vi "Visualizacion_NEW.vi"() -> ()   [LabVIEW 2021]
uses:
  <vilib>/Modbus/master/Modbus Master.lvclass
  <vilib>/Modbus/master/Create Master Instance (TCP).vi
panel:
  out "MEAN (T)":sgl format="%0.2f"
  out "Peltiers enable":bool
  out "Program Status":bool
  out "SP (T)":sgl
  out "Segmento_temp":u16
  in  "?":T1(tab)
  in  "?":T2(tab)
  out "TEMPERATURA MEDIA":dynamicdata(graph)
  out "ALL TOGETHER":dynamicdata(graph)
  out "VALVULA 1 Y BOBINA 1":dynamicdata(graph)
  out "VALVULA 2 Y BOBINA 2":dynamicdata(graph)
  out "VALVULA 3 Y BOBINA 3":dynamicdata(graph)
  out "VALVULA 4 Y BOBINA 4":dynamicdata(graph)
  out "VALVULA 5  Y BOBINA 5":dynamicdata(graph)
  out "VALVULA 6 Y BOBINA 6":dynamicdata(graph)
  out "VALVULA 7 Y BOBINA 7":dynamicdata(graph)
  out "VALVULA 8 Y PELTIER 8":dynamicdata(graph)
  out "Camara climatica":dynamicdata(graph)
  out "current time":timestamp
  out "W1.16":bool
  out "W1.15":bool
  out "W1.11":bool
  out "1.10":bool
  out "W1.14":bool
  out "W1.13":bool
  out "W1.12":bool
  out "W1.1":bool
  out "W2":bool
  out "W3":bool
  out "W4":bool
  out "W1.2":bool
  out "W1.3":bool
  out "W1.6":bool
  out "W1.5":bool
  out "W1.4":bool
  out "W1.9":bool
  out "W1.8":bool
  out "W1.7":bool
  out "warnings table":T3(array[cluster]) {"Time Stamp" format="%<%.3X %x>T"}
  in  "Reset":bool
  out "Comunicacion Modbus":errorcluster
  in  "Digital Input Bitron Simulation":bool
  in  "Pelt ºC/min":dbl=2.5
  in  "Cam ºC/min":dbl=2.2
  in  "Tiempo máximo de ciclo(min)":dbl=90.0
  in  "Setpoint corte frío(ºC)":dbl=-30.0
  in  "Setpoint Frío(ºC)":dbl=-40.0
  in  "Setpoint peltiers(ºC)":dbl=85.0
  in  "Tiempo estabilidad de Frío(min)":dbl=15.0
  in  "Tiempo mínimo de ciclo(min)":dbl=70.0
  in  "Setpoint calor corte rampa(ºC)":dbl=51.0
  in  "T ciclo (Bitron FSM Sim)":dbl=90.0
  in  "Setpoint calor cam":dbl=55.0
  in  "Save Parameters":bool
  in  "PWM 4(SP)":u16
  in  "PWM 3(SP) 2":u16
  in  "PWM 2(SP) 2":u16
  in  "PWM 1(SP) 2":u16
  in  "PWM 8(SP)":u16
  in  "PWM 7(SP)":u16
  in  "PWM 6(SP)":u16
  in  "PWM 5(SP)":u16
  in  "Test PWM (%)":bool
  in  "Conf PIDs":bool
  in  "TestPID 8(ºC)":u16
  in  "TestPID 4(ºC)":u16
  in  "TestPID3(ºC)":u16
  in  "TestPID 2(ºC)":u16
  in  "TestPID 1(ºC)":u16
  in  "TestPID 5(ºC)":u16
  in  "TestPID 6(ºC)":u16
  in  "TestPID 7(ºC)":u16
  out "Temp Man 2":sgl
  out "PWM 1(SP)":u16
  out "Temp Man 3":sgl format="%#.2g"
  out "Temp Man 1":sgl format="%#.2g"
  out "Temp Man 4":sgl
  out "PWM 2(SP)":u16
  out "Temp Man 5":sgl format="%#.2g"
  out "PWM 3(SP)":u16
  out "PWM 4(SP)":u16
  out "Temp Man 6":sgl
  out "Temp Man 7":sgl format="%#.2g"
  out "Temp Man 8":sgl
  out "PWM 6(SP)":u16
  out "PWM 7(SP)":u16
  out "PWM 5(SP)":u16
  out "PWM 8(SP)":u16
  out "Temp bob 1":sgl
  out "Temp bob 2":sgl
  out "Temp bob 3":sgl format="%#.2g"
  out "Temp bob 6":sgl
  out "Temp bob 7":sgl format="%#.2g"
  out "Temp bob 8":sgl
  in  "Enable PI 5":bool
  in  "Enable PI 6":bool=TRUE
  in  "Enable PI 7":bool
  in  "Enable PI 8":bool
  out "Temp bob 5":sgl format="%#.2g"
  in  "Descarte Media Temps":u16=1 max=3 step=1
  out "Temp bob 4":sgl
  in  "Enable PI 1":bool
  in  "Enable PI 2":bool
  in  "Enable PI 3":bool
  in  "Enable PI 4":bool=TRUE
  in  "Test PID (ºC)":bool
  in  "Tiempo de guardado":u32=600
  out "data to be saved":dbl[][](array[numeric])
  out "Guardando en disco":bool
  out "array w/ subset deleted":dbl[][](array[numeric])
  out "size(s)":i32
  out "W to save":string[][](array[string])
  in  "Warning saved":bool
  in  "Tiempo/dato (s)":u32=1
  out "DO H2 Lab":bool
  in  "Guardar datos":bool=TRUE
  out "senal_bitron":bool
  in  "Stop Control Program":bool
  out "Coils write":bool[](array[boolean])
  out "Int values":u16[](array[numeric])
  out "SGL values":sgl[](array[numeric])
  out "coil values":bool[](array[boolean])
  out "ComunicacionCRIO":bool
  in  "run_program":bool
  out "Setpoint_temp_write":dbl
  out "Setpoint_hum_write":dbl
  out "Temperatura Camara":dbl
  out "Humedad relativa (HR)":dbl
  in  "Pause_Entrar_camara":bool
  in  "Pause":bool
  in  "stop":bool
  in  "Tab Control":T4(tab)
  out "T Man 5":dbl(slide) scale=-45.0..90.0
  out "T Man 1":dbl(slide) scale=-45.0..90.0
  out "T Man 2":dbl(slide) scale=-45.0..90.0
  out "T Man 3":dbl(slide) scale=-45.0..90.0
  out "T Man 4":dbl(slide) scale=-45.0..90.0
  out "T Man 6":dbl(slide) scale=-45.0..90.0
  out "T Man 7":dbl(slide) scale=-45.0..90.0
  out "T Man 8":dbl(slide) scale=-45.0..90.0
  out "T bob 5":dbl(slide) scale=-45.0..95.0
  out "T bob 1":dbl(slide) scale=-45.0..95.0
  out "T bob 2":dbl(slide) scale=-45.0..95.0
  out "T bob 3":dbl(slide) scale=-45.0..95.0
  out "T bob 4":dbl(slide) scale=-45.0..95.0
  out "T bob 6":dbl(slide) scale=-45.0..95.0
  out "T bob 7":dbl(slide) scale=-45.0..95.0
  out "T bob 8":dbl(slide) scale=-45.0..95.0
  # "Control Programa Principal"
  # "Cámara climática"
  # "ºC"
  # "ºC"
  # "%"
  # "%"
  # "Simulación señal Bitron"
  # "ºC"
  # "HR"
  # "TempCC"
  # "SP_HR"
  # "SP_TempCC"
  # "Mean T"
  # "Warnings y Errores"
  # "Parametros y configuracion para la curva de ciclado"
  # "ºC"
  # "ºC"
  # "VALVE 4"
  # "VALVE 8"
  # "%"
  # "%"
  # "ºC"
  # "ºC"
  # "ºC"
  # "ºC"
  # "VALVE 3"
  # "%"
  # "%"
  # "VALVE 7"
  # "ºC"
  # "ºC"
  # "ºC"
  # "ºC"
  # "VALVE 2"
  # "%"
  # "%"
  # "VALVE 6"
  # "ºC"
  # "ºC"
  # "ºC"
  # "ºC"
  # "VALVE 1"
  # "%"
  # "%"
  # "VALVE 5"
  # "ºC"
  # "ºC"
  # "1 Dato\n----------------"
  # "Frecuencia de guardado:"
  # "s"
  # "s"
  # "T Manifolds:"
  # "1               2               3               4               5               6               7               8"
  # "T Bobinas:"
  # "1               2               3               4               5                 6               7               8"
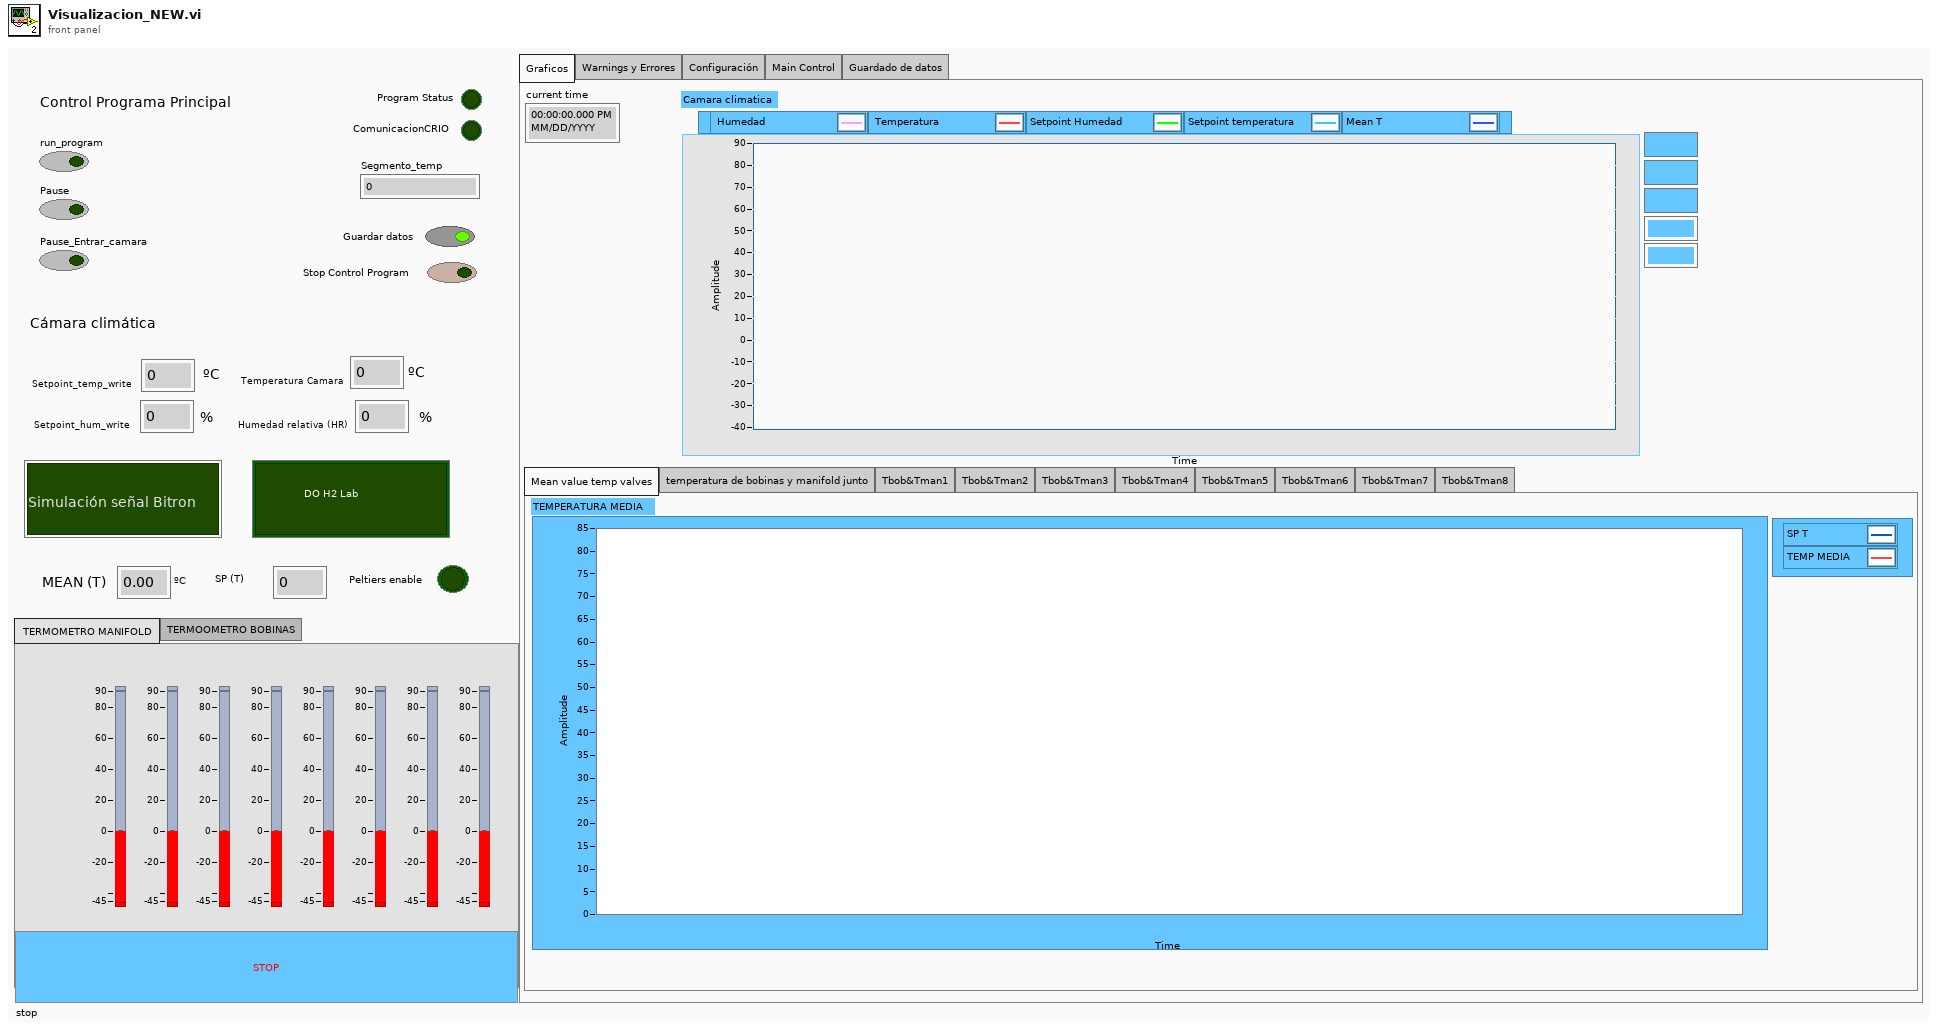
[diagram p1: front panel]
types:
  T1 = enum32{"Graficos", "Warnings y Errores", "Configuración", "Main Control", "Guardado de datos"}
  T2 = enum32{"Mean value temp valves", "temperatura de bobinas y manifold junto", "Tbob&Tman1", "Tbob&Tman2", "Tbob&Tman3", "Tbob&Tman4", "Tbob&Tman5", "Tbob&Tman6", "Tbob&Tman7", "Tbob&Tman8"}
  T3 = cluster{"Time Stamp":timestamp, "Descripcion":string, "Numeric":i32}[]
  T4 = enum32{"TERMOMETRO MANIFOLD ", "TERMOOMETRO BOBINAS"}
  T5 = enum8{"Enabled", "Disabled", "Disabled and Grayed Out"}
  T6 = enum16{"open", "open or create", "create or replace", "create", "open (read-only)"}
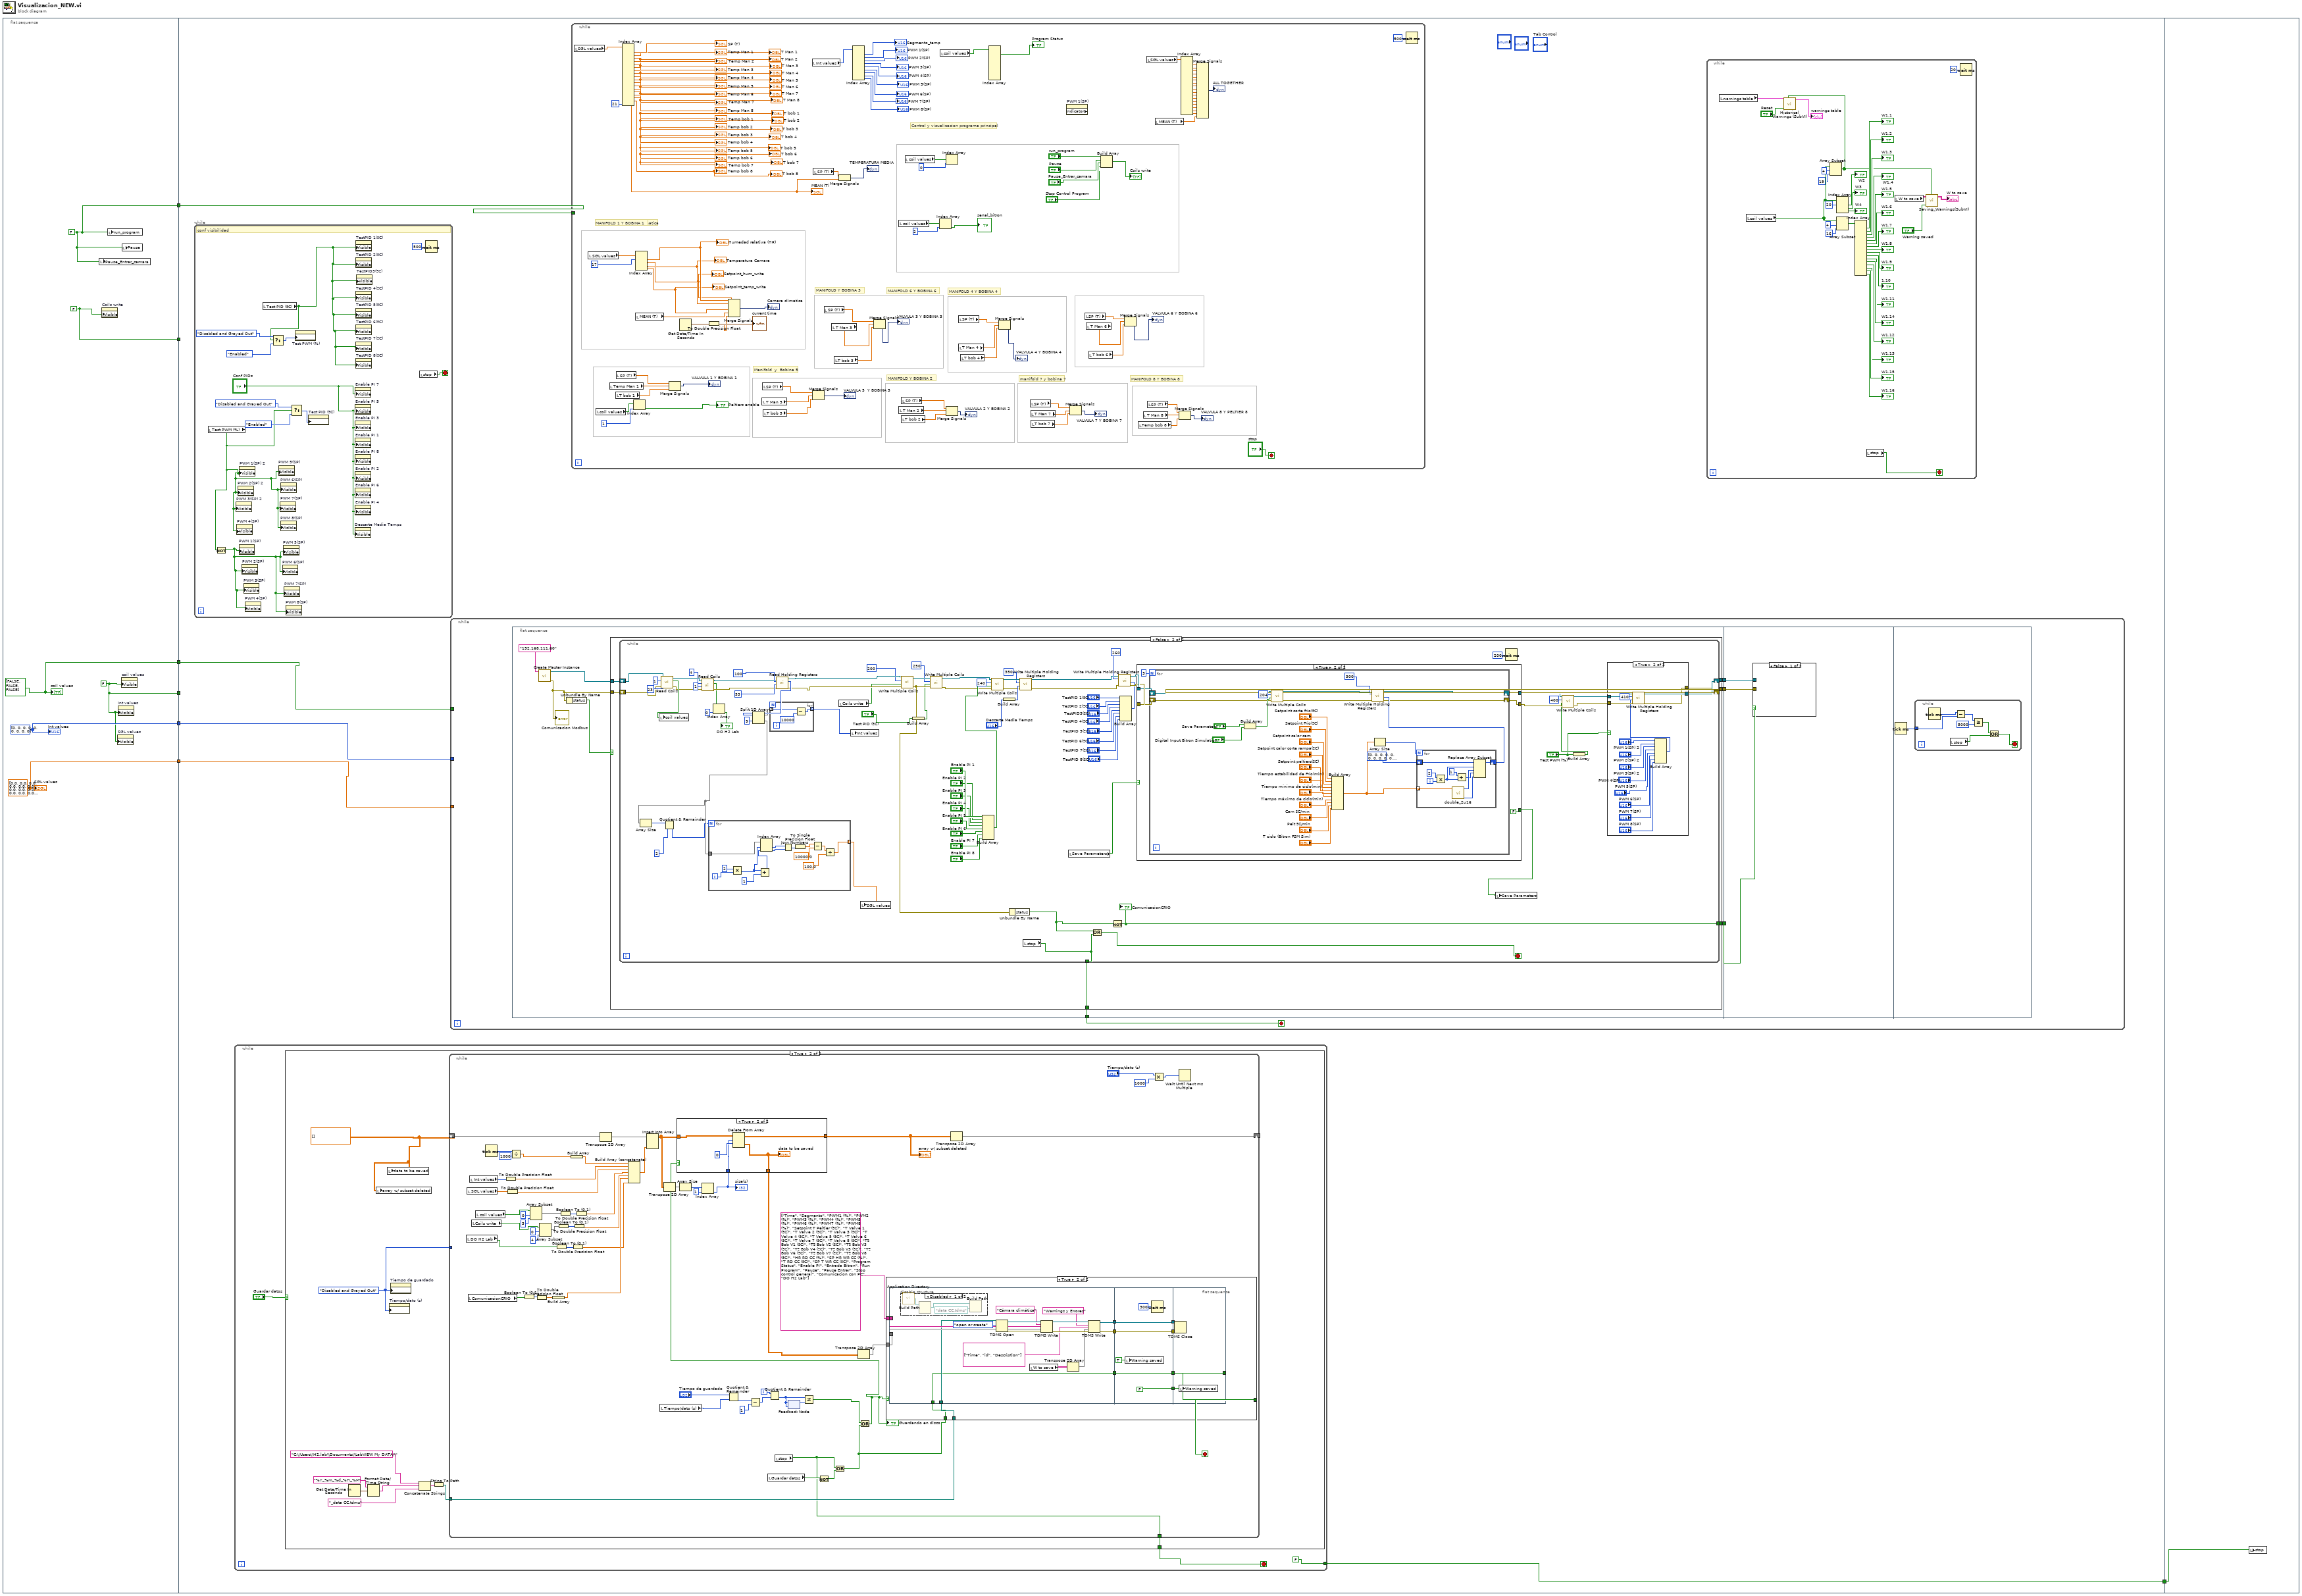
[diagram p0: block diagram]
diagram:
  n1 = flat-sequence {
    tunnel: [w13] -> w7
    tunnel: [w12] -> w6
    tunnel: [w11] -> w5
    tunnel: [w10] -> w4
    tunnel: [w8] -> w2
    tunnel: [w9] -> w1
    tunnel: w7 -> [w18]
    tunnel: w6 -> [w17]
    tunnel: w5 -> [w16]
    tunnel: w4 -> [w15]
    tunnel: [w14] -> w3
    tunnel: w2 -> [_]
    tunnel: w1 -> [_]
    tunnel: w3 -> [w501]
    frame #0 {
      w9 = FALSE ("Visible")
      w8 = FALSE ("Visible")
      w11 = sgl[] [0.0, 0.0, 0.0, 0.0, 0.0, 0.0, 0.0, 0.0, 0.0, 0.0, 0.0, 0.0, 0.0, 0.0, 0.0, 0.0, 0.0, 0.0, 0.0, 0.0, 0.0] ("SGL values")
      w12 = u16[] [0, 0, 0, 0, 0, 0, 0, 0, 0] ("Int values")
      w10 = FALSE ("run_program")
      w13 = bool[] [FALSE, FALSE, FALSE] ("coil values")
      n2 = local write "Pause_Entrar_camara"(w10) -> ()
      n3 = property on="Coils write" class="Arr (strict)"("Visible"=w9) -> ()  [unwired: 2 in, 2 out]
      n4 = local write "run_program"(w10) -> ()
      n5 = property on="SGL values" class="Arr (strict)"("Visible"=w8) -> ()  [unwired: 2 in, 2 out]
      n6 = property on="Int values" class="Arr (strict)"("Visible"=w8) -> ()  [unwired: 2 in, 2 out]
      n7 = property on="coil values" class="Arr (strict)"("Visible"=w8) -> ()  [unwired: 2 in, 2 out]
      n8 = local write "Pause"(w10) -> ()
      "coil values" <- w13
      "Int values" <- w12
      "SGL values" <- w11
    }
    frame #1 {
      n9 = while {
        stop <- w30 stop-if-true
        # "conf visibilidad"
        n10 = local read "Test PWM (%)"() -> (w19:bool)
        n11 = Not(x=w19) -> (.not. x?=w27:bool)
        n12 = property on="PWM 3(SP) 2" class="DigNum (strict)"("Visible"=w19) -> ()  [unwired: 2 in, 2 out]
        n13 = property on="PWM 4(SP)" class="DigNum (strict)"("Visible"=w19) -> ()  [unwired: 2 in, 2 out]
        n14 = property on="PWM 2(SP) 2" class="DigNum (strict)"("Visible"=w19) -> ()  [unwired: 2 in, 2 out]
        n15 = property on="PWM 1(SP)" class="DigNum (strict)"("Visible"=w27) -> ()  [unwired: 2 in, 2 out]
        n16 = property on="PWM 1(SP) 2" class="DigNum (strict)"("Visible"=w19) -> ()  [unwired: 2 in, 2 out]
        n17 = property on="PWM 2(SP)" class="DigNum (strict)"("Visible"=w27) -> ()  [unwired: 2 in, 2 out]
        n18 = property on="PWM 3(SP)" class="DigNum (strict)"("Visible"=w27) -> ()  [unwired: 2 in, 2 out]
        n19 = property on="PWM 4(SP)" class="DigNum (strict)"("Visible"=w27) -> ()  [unwired: 2 in, 2 out]
        n20 = local read "Test PID (ºC)"() -> (w23:bool)
        n21 = Select(t=T5."Disabled and Grayed Out" ("Disabled"), s=w23, f=T5."Enabled" ("Disabled")) -> (s? t:f=w24:T5)
        n22 = property on="PWM 5(SP)" class="DigNum (strict)"("Visible"=w19) -> ()  [unwired: 2 in, 2 out]
        n23 = property on="PWM 7(SP)" class="DigNum (strict)"("Visible"=w19) -> ()  [unwired: 2 in, 2 out]
        n24 = property on="PWM 6(SP)" class="DigNum (strict)"("Visible"=w19) -> ()  [unwired: 2 in, 2 out]
        n25 = property on="PWM 8(SP)" class="DigNum (strict)"("Visible"=w19) -> ()  [unwired: 2 in, 2 out]
        n26 = property on="PWM 6(SP)" class="DigNum (strict)"("Visible"=w27) -> ()  [unwired: 2 in, 2 out]
        n27 = property on="PWM 5(SP)" class="DigNum (strict)"("Visible"=w27) -> ()  [unwired: 2 in, 2 out]
        n28 = property on="PWM 7(SP)" class="DigNum (strict)"("Visible"=w27) -> ()  [unwired: 2 in, 2 out]
        n29 = property on="PWM 8(SP)" class="DigNum (strict)"("Visible"=w27) -> ()  [unwired: 2 in, 2 out]
        n30 = Select(t=T5."Disabled and Grayed Out" ("Disabled"), s=w19, f=T5."Enabled" ("Disabled")) -> (s? t:f=w20:T5)
        n31 = property on="Test PWM (%)" class="Bool (strict)"("DisabledEnum"=w24) -> ()  [unwired: 2 in, 2 out]
        n32 = property on="Test PID (ºC)" class="Bool (strict)"("DisabledEnum"=w20) -> ()  [unwired: 2 in, 2 out]
        n33 = property on="Descarte Media Temps" class="DigNum (strict)"("Visible"="Conf PIDs") -> ()  [unwired: 2 in, 2 out]
        n34 = property on="Enable PI 7" class="Bool (strict)"("Visible"="Conf PIDs") -> ()  [unwired: 2 in, 2 out]
        n35 = property on="Enable PI 5" class="Bool (strict)"("Visible"="Conf PIDs") -> ()  [unwired: 2 in, 2 out]
        n36 = property on="Enable PI 3" class="Bool (strict)"("Visible"="Conf PIDs") -> ()  [unwired: 2 in, 2 out]
        n37 = property on="Enable PI 1" class="Bool (strict)"("Visible"="Conf PIDs") -> ()  [unwired: 2 in, 2 out]
        n38 = property on="Enable PI 8" class="Bool (strict)"("Visible"="Conf PIDs") -> ()  [unwired: 2 in, 2 out]
        n39 = property on="Enable PI 2" class="Bool (strict)"("Visible"="Conf PIDs") -> ()  [unwired: 2 in, 2 out]
        n40 = property on="Enable PI 6" class="Bool (strict)"("Visible"="Conf PIDs") -> ()  [unwired: 2 in, 2 out]
        n41 = property on="Enable PI 4" class="Bool (strict)"("Visible"="Conf PIDs") -> ()  [unwired: 2 in, 2 out]
        n42 = property on="TestPID 1(ºC)" class="DigNum (strict)"("Visible"=w23) -> ()  [unwired: 2 in, 2 out]
        n43 = property on="TestPID 2(ºC)" class="DigNum (strict)"("Visible"=w23) -> ()  [unwired: 2 in, 2 out]
        n44 = property on="TestPID 4(ºC)" class="DigNum (strict)"("Visible"=w23) -> ()  [unwired: 2 in, 2 out]
        n45 = property on="TestPID 5(ºC)" class="DigNum (strict)"("Visible"=w23) -> ()  [unwired: 2 in, 2 out]
        n46 = property on="TestPID 6(ºC)" class="DigNum (strict)"("Visible"=w23) -> ()  [unwired: 2 in, 2 out]
        n47 = property on="TestPID 7(ºC)" class="DigNum (strict)"("Visible"=w23) -> ()  [unwired: 2 in, 2 out]
        n48 = property on="TestPID 8(ºC)" class="DigNum (strict)"("Visible"=w23) -> ()  [unwired: 2 in, 2 out]
        n49 = property on="TestPID3(ºC)" class="DigNum (strict)"("Visible"=w23) -> ()  [unwired: 2 in, 2 out]
        n50 = local read "stop"() -> (w30:bool)
        n51 = Wait (ms)(milliseconds to wait=u32 500) -> ()  [unwired: 1 out]
      }
      n52 = while {
        tunnel: [FALSE ("stop Control General")] -> w14
        stop <- w67 stop-if-true
        n53 = case shown="True" "Guardar datos" {
          tunnel: [w70 w73] -> w67
          frame False {
            w69 = T5."Enabled" ("Disabled")
            n54 = property on="Tiempo/dato (s)" class="DigNum (strict)"("DisabledEnum"=w69) -> ()  [unwired: 2 in, 2 out]
            n55 = property on="Tiempo de guardado" class="DigNum (strict)"("DisabledEnum"=w69) -> ()  [unwired: 2 in, 2 out]
            n56 = local read "stop"() -> (w70:bool)
            n57 = Wait Until Next ms Multiple(millisecond multiple=u32 1000 ("milliseconds to wait")) -> ()  [unwired: 1 out]
          }
          frame True {
            w72 = T5."Disabled and Grayed Out" ("Disabled")
            w81 = dbl[][] []
            n58 = Get Date/Time In Seconds() -> (seconds since 1Jan1904=w80:timestamp)
            n59 = Format Date/Time String(time format string (%c)="%Y_%m_%d_%H_%M", seconds (now)=w80) -> (date/time string=w77:string)  [unwired: 1 in]
            n60 = local write "array w/ subset deleted"(w81) -> ()
            n61 = local write "data to be saved"(w81) -> ()
            n62 = property on="Tiempo/dato (s)" class="DigNum (strict)"("DisabledEnum"=w72) -> ()  [unwired: 2 in, 2 out]
            n63 = property on="Tiempo de guardado" class="DigNum (strict)"("DisabledEnum"=w72) -> ()  [unwired: 2 in, 2 out]
            n64 = Concatenate Strings("C:\\Users\\H2.lab\\Documents\\LabVIEW My DATA\\" ("string"), w77, "_data CC.tdms" ("string")) -> (w78:string)
            n65 = String To Path(string=w78) -> (path=w75:path)
            n66 = while {
              shift-right: [w131] -> _
              shift-left: w81 -> [w134]
              tunnel: w75 -> [w123]
              tunnel: [w101] -> w73
              tunnel: w72 -> [_]
              i -> [w138]
              stop <- w105 stop-if-true
              n67 = local read "DO H2 Lab"() -> (w99:bool)
              n68 = local read "SGL values"() -> (w121:sgl[])
              n69 = local read "ComunicacionCRIO"() -> (w107:bool)
              n70 = local read "Int values"() -> (w122:u16[])
              n71 = local read "Coils write"() -> (w93:bool[])
              n72 = local read "coil values"() -> (w97:bool[])
              n73 = Tick Count (ms)() -> (millisecond timer value=w125:u32)
              n74 = To Double Precision Float(number=w122) -> (double precision float=w120:dbl[])
              n75 = To Double Precision Float(number=w121) -> (double precision float=w119:dbl[])
              n76 = Divide(x=w125, y=u32 1000) -> (x/y=w118:dbl)
              n77 = Boolean To (0,1)(Boolean=w107) -> (0, 1=w114:i16)
              n78 = Array Subset(array=w97, index=0, length=3) -> (w96:bool[])
              n79 = To Double Precision Float(number=w114) -> (double precision float=w113:dbl)
              n80 = Array Subset(array=w93, index=0, length=4) -> (w90:bool[])
              n81 = Build Array(w113) -> (w110:dbl[])
              n82 = Boolean To (0,1)(Boolean=w99) -> (0, 1=w100:i16)
              n83 = Boolean To (0,1)(Boolean=w90) -> (0, 1=w109:i16[])
              n84 = Boolean To (0,1)(Boolean=w96) -> (0, 1=w116:i16[])
              n85 = Build Array(w118) -> (w117:dbl[])
              n86 = To Double Precision Float(number=w100) -> (double precision float=w98:dbl)
              n87 = To Double Precision Float(number=w109) -> (double precision float=w108:dbl[])
              n88 = To Double Precision Float(number=w116) -> (double precision float=w115:dbl[])
              n89 = Transpose 2D Array(2D array=w134) -> (transposed array=w133:dbl[][])
              n90 = Build Array (concatenate)(w117, w120, w119, w115, w108, w110, w98) -> (w139:dbl[])
              n91 = Insert Into Array(array=w133, new element=w139) -> (w136:dbl[][])  [unwired: 2 in]
              n92 = local read "Tiempo/dato (s)"() -> (w85:u32)
              n93 = Transpose 2D Array(2D array=w136) -> (transposed array=w130:dbl[][])
              n94 = Array Size(array=w130) -> (size(s)=w129:i32[])
              n95 = Index Array(array=w129, index=1) -> (element=w128:i32)
              "size(s)" <- w128
              n96 = Quotient & Remainder(x="Tiempo de guardado", y=w85) -> (floor(x/y)=w84:u32)  [unwired: 1 out]
              n97 = Subtract(x=w84, y=u32 1) -> (x-y=w83:u32)
              n98 = local read "Guardar datos"() -> (w104:bool)
              n99 = Quotient & Remainder(x=w138, y=w83) -> (floor(x/y)=w135:u32)  [unwired: 1 out]
              n100 = local read "stop"() -> (w101:bool)
              n101 = feedback-in #1(w135) -> ()
              n102 = feedback #1(w135) -> (w137:u32)
              n103 = Not Equal?(x=w135, y=w137) -> (x != y?=w106:bool)
              n104 = Not(x=w104) -> (.not. x?=w103:bool)
              n105 = Or(x=w101, y=w103) -> (x .or. y?=w102:bool)
              n106 = Or(x=w106, y=w102) -> (x .or. y?=w112:bool)
              "Guardando en disco" <- w112
              n107 = case shown="True" w112 {
                tunnel: w136 -> [w142 w145]
                tunnel: [w142 w147] -> w132
                tunnel: w128 -> [_ w144]
                tunnel: [dbl[][] [] w143] -> w111
                frame False {
                }
                frame True {
                  n108 = Delete From Array(array=w145, length=w144, index (row)=0) -> (deleted portion=w143:dbl[][], array with subset deleted=w147:dbl[][])  [unwired: 1 in]
                  "data to be saved" <- w143
                }
              }
              "array w/ subset deleted" <- w132
              n109 = Transpose 2D Array(2D array=w111) -> (transposed array=w126:dbl[][])
              n110 = case shown="True" w112 {
                tunnel: string[] ["Time", "Segmento", "PWM1 (%)", "PWM2 (%)", "PWM3 (%)", "PWM4 (%)", "PWM5 (%)", "PWM6 (%)", "PWM7 (%)", "PWM8 (%)", "Setpoint T Peltier (ºC)", "T Valve 1 (ºC)", "T Valve 2 (ºC)", "T Valve 3 (ºC)", "T Valve 4 (ºC)", "T Valve 5 (ºC)", "T Valve 6 (ºC)", "T Valve 7 (ºC)", "T Valve 8 (ºC)", "Tª Bob V1 (ºC)", "Tª Bob V2 (ºC)", "Tª Bob V3 (ºC)", "Tª Bob V4 (ºC)", "Tª Bob V5 (ºC)", "Tª Bob V6 (ºC)", "Tª Bob V7 (ºC)", "Tª Bob V8 (ºC)", "HR RD CC (%)", "SP HR WR CC (%)", "T RD CC (ºC)", "SP T WR CC (ºC)", "Program Status", "Enable PI", "Entrada Bitron", "Run Program", "Pause", "Pause Entrar", "Stop control general", "Comunicacion con PC", "DO H2 Lab"] -> [_ w160]
                tunnel: w126 -> [_ w159]
                tunnel: w123 -> [_ w158]
                tunnel: w102 -> [_ w157]
                tunnel: [FALSE ("STOP ALL") w156] -> w105